vi "TLB Native Dynamic Events ver 0.25.vi"() -> ()   [LabVIEW 2018] (continued)
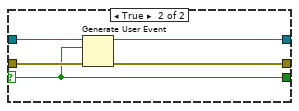
[diagram p2: hidden frame]
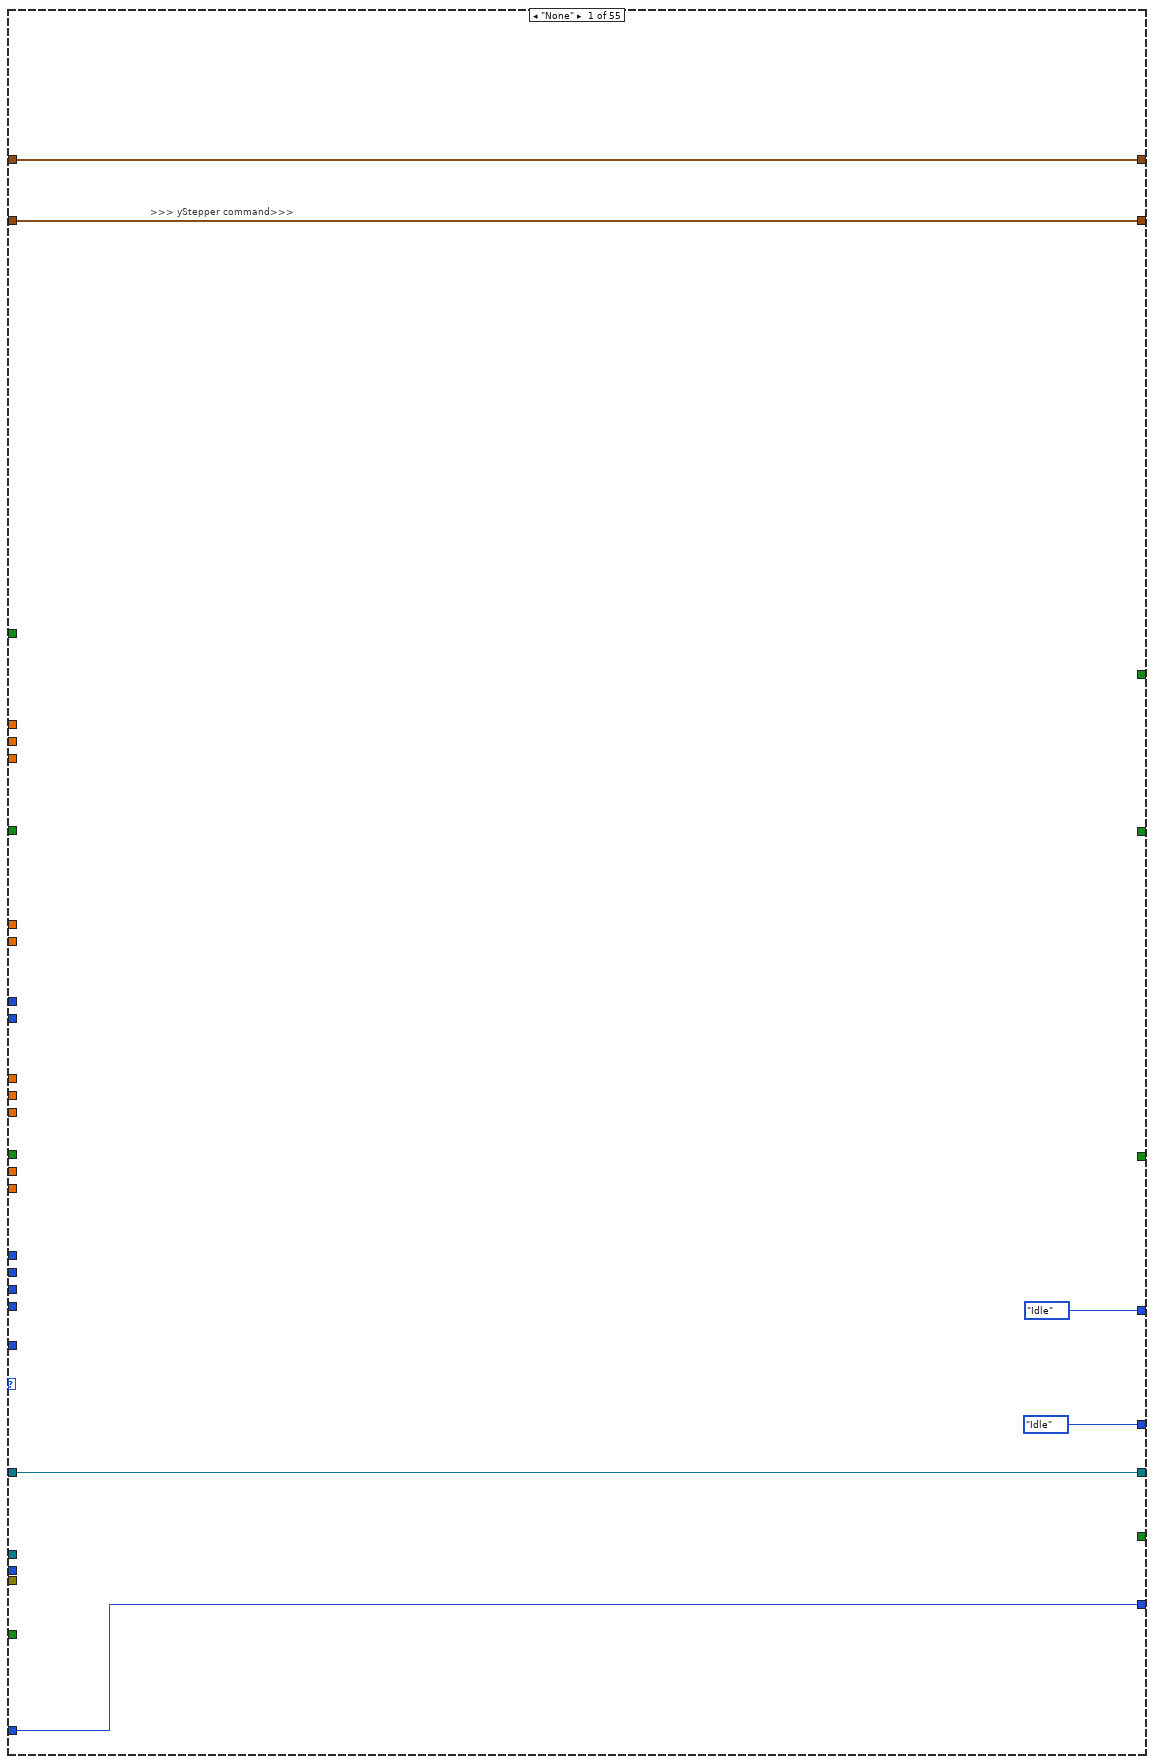
[diagram p5: hidden frame]
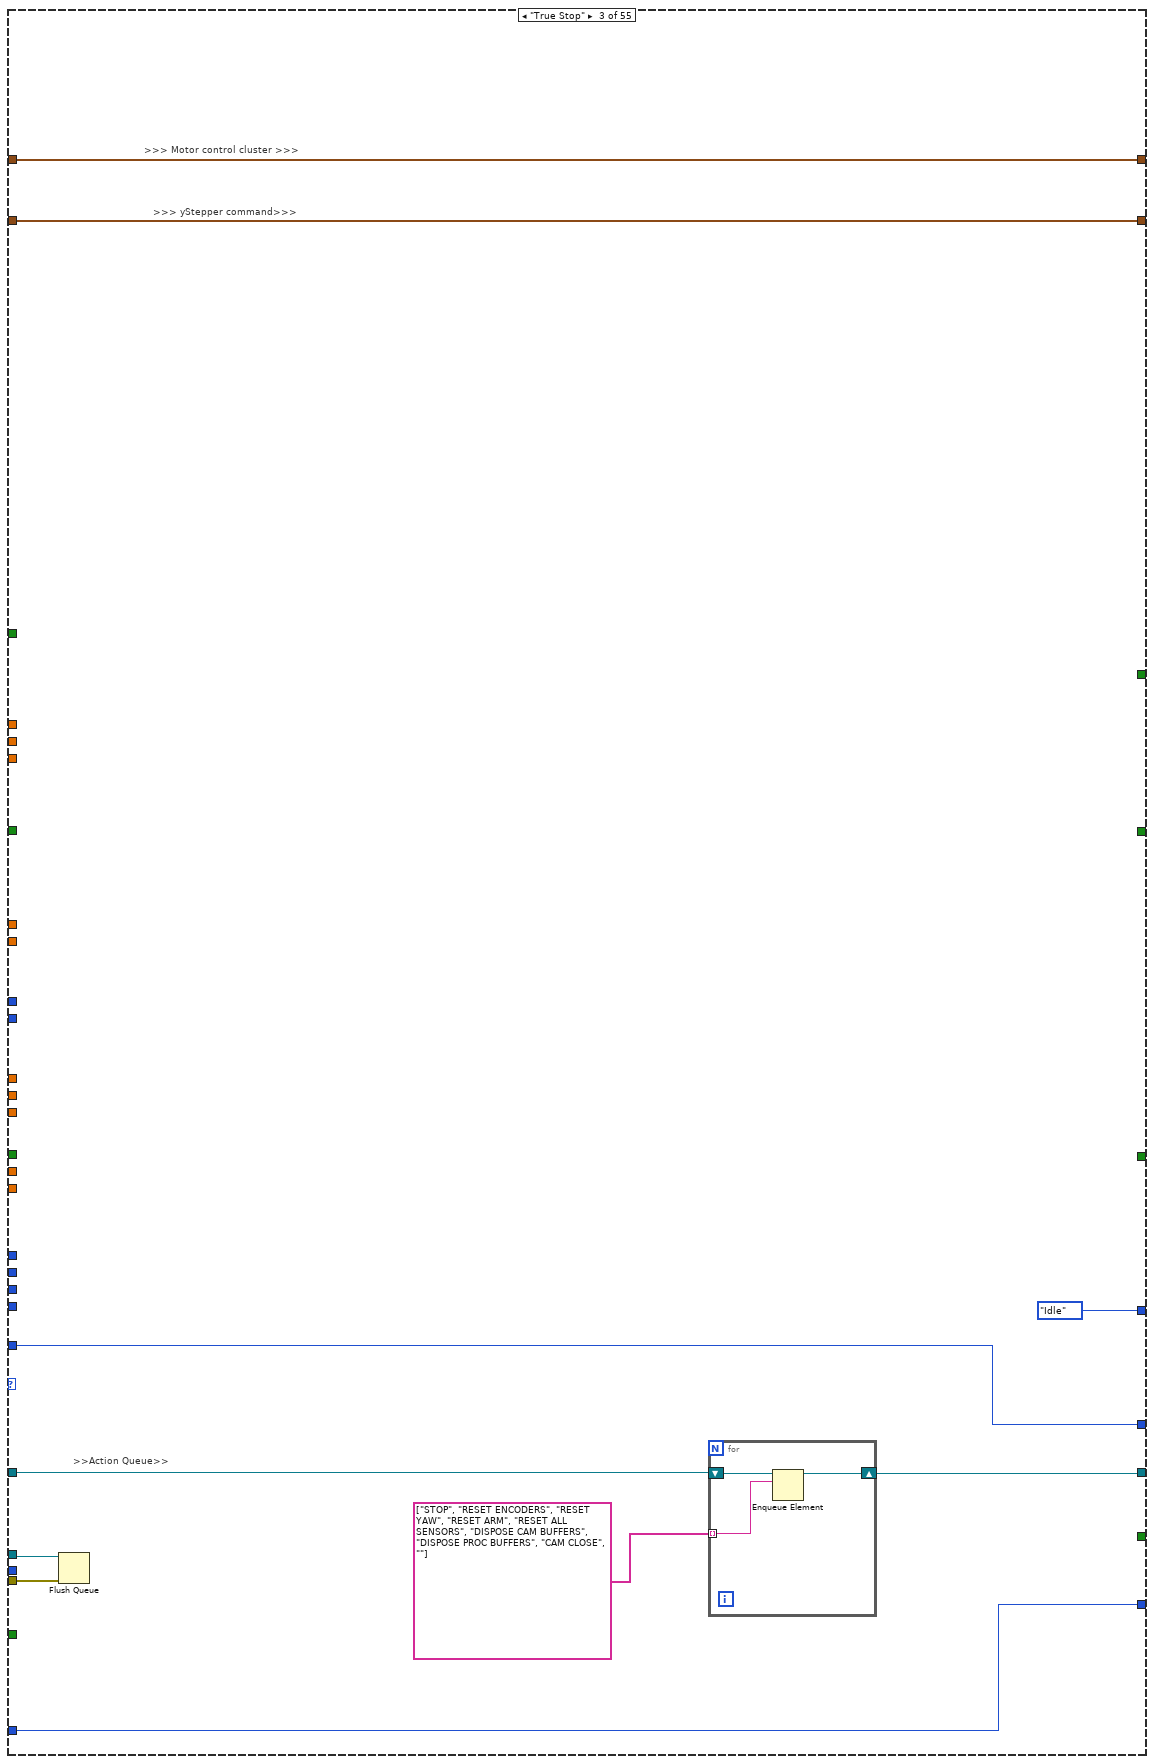
[diagram p6: hidden frame]
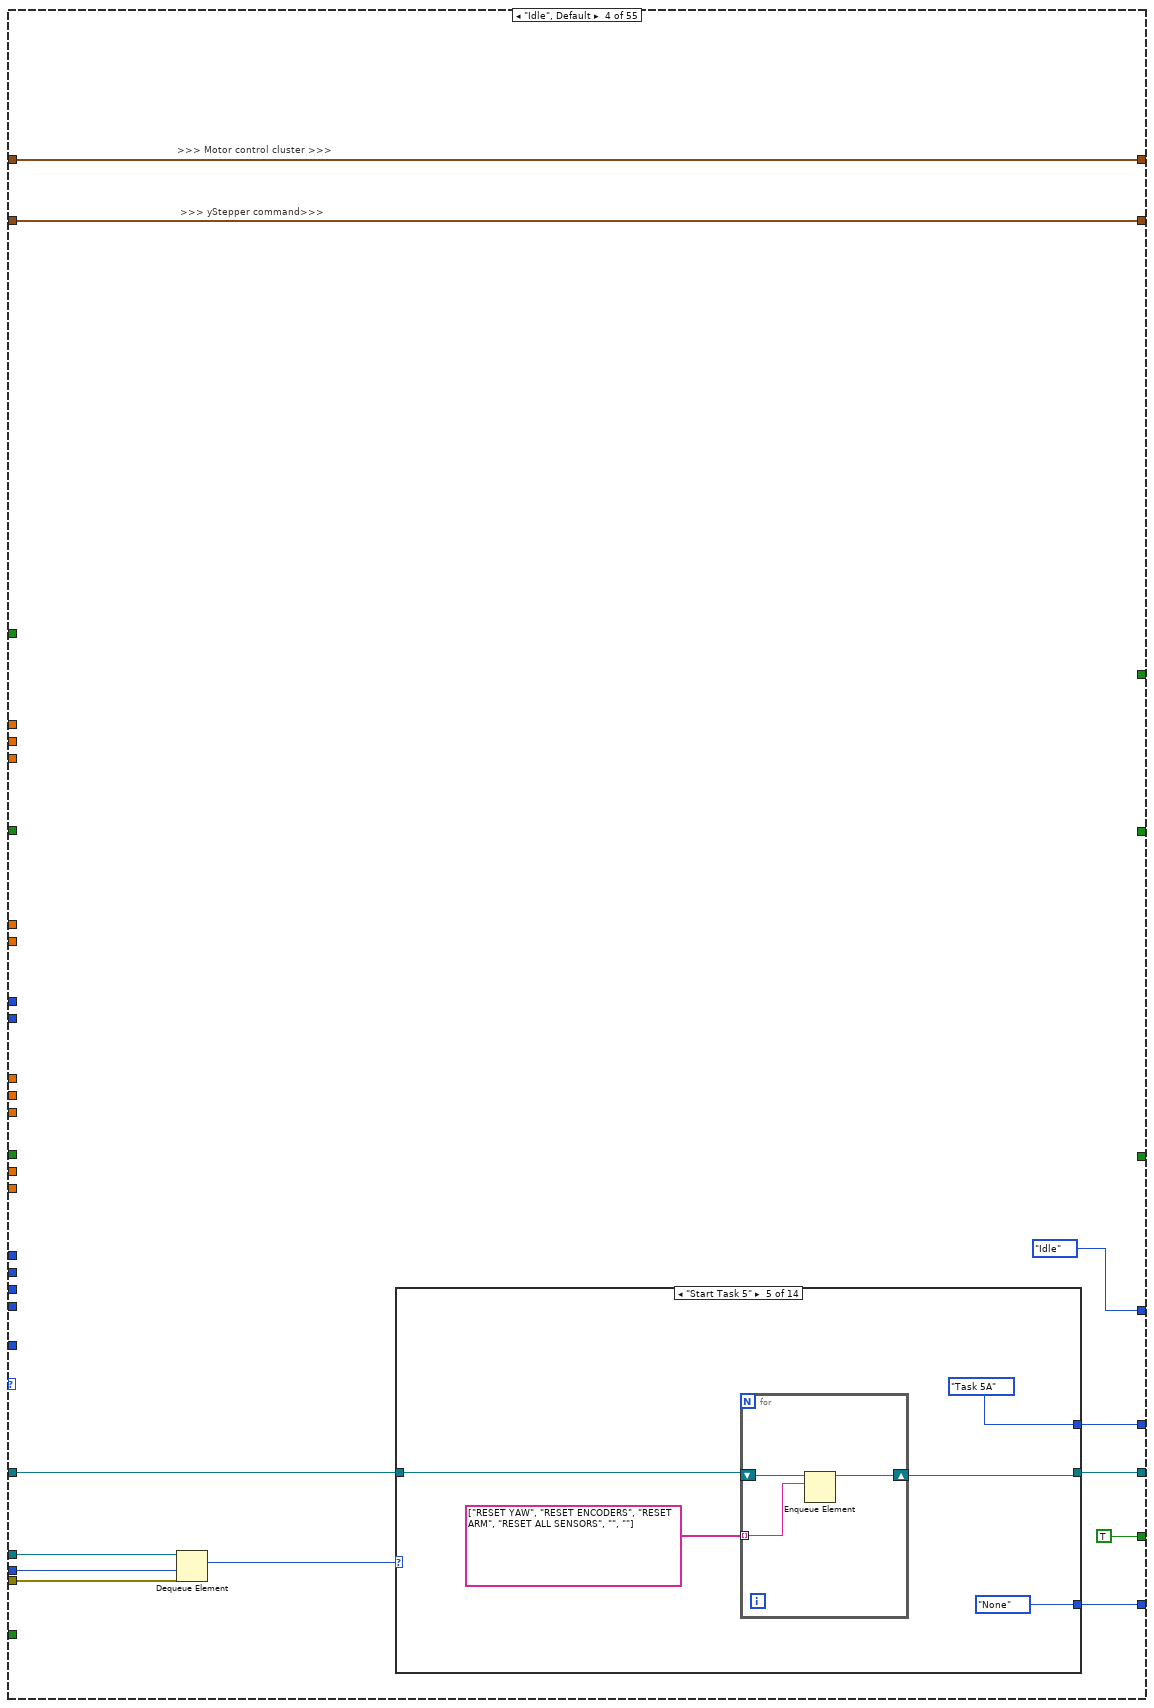
[diagram p7: hidden frame]
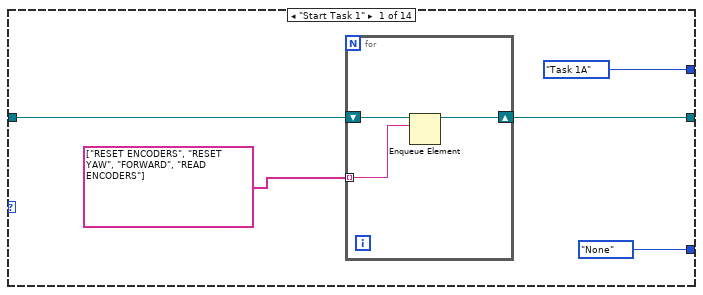
[diagram p8: hidden frame]
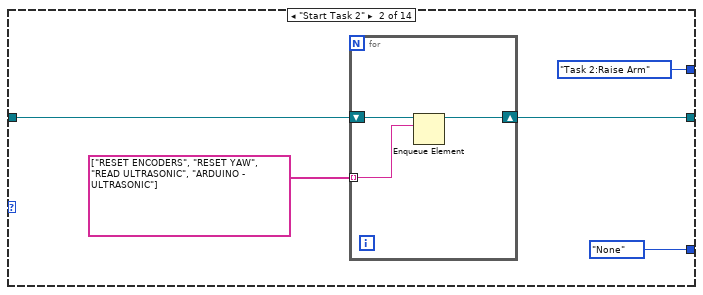
[diagram p9: hidden frame]
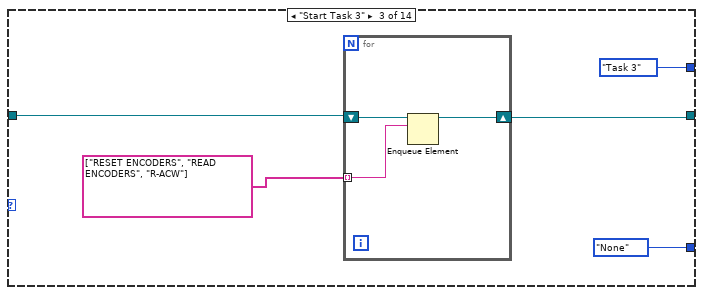
[diagram p10: hidden frame]
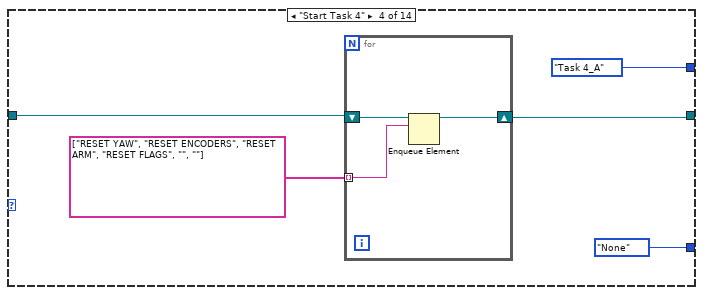
[diagram p11: hidden frame]
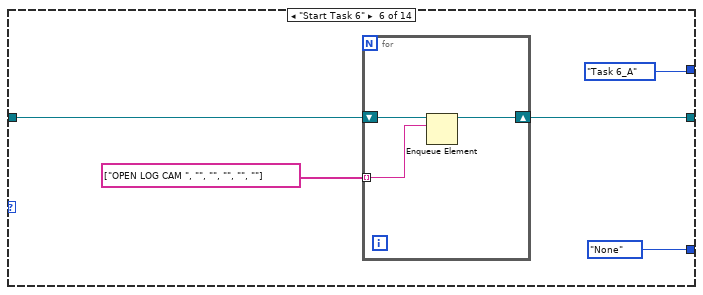
[diagram p12: hidden frame]
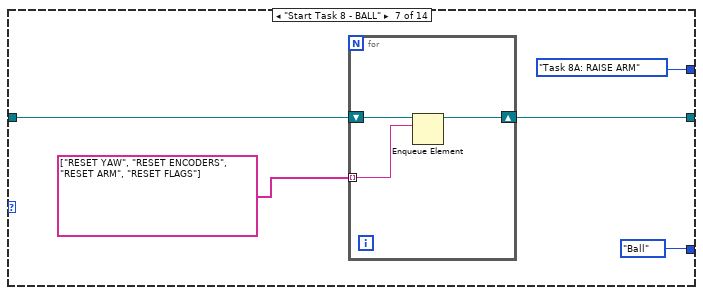
[diagram p13: hidden frame]
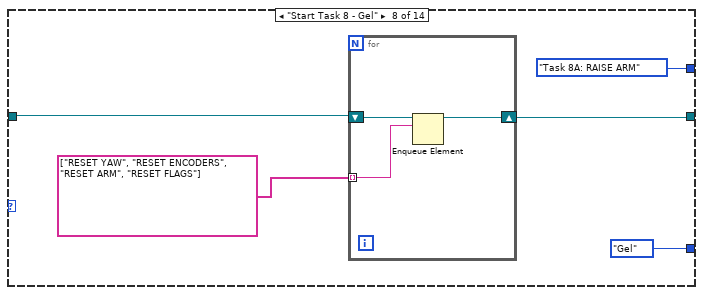
[diagram p14: hidden frame]
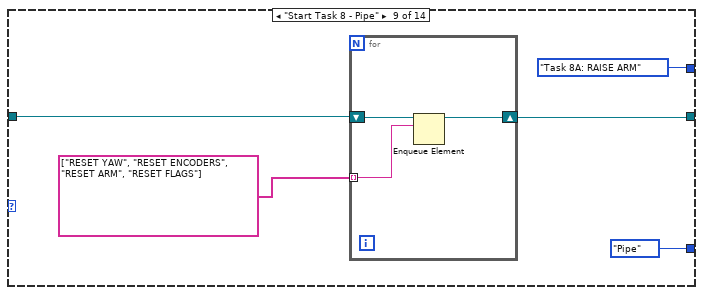
[diagram p15: hidden frame]
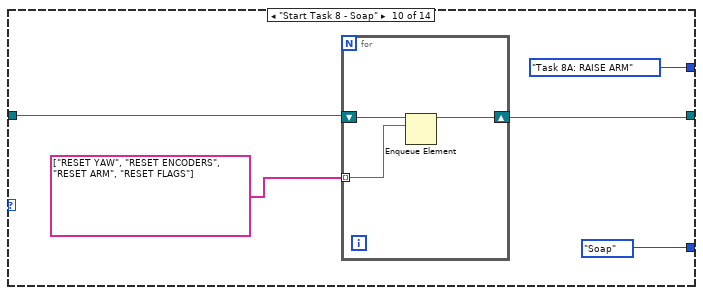
[diagram p16: hidden frame]
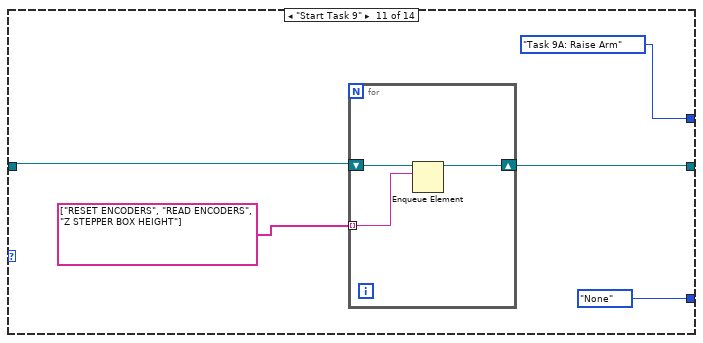
[diagram p17: hidden frame]
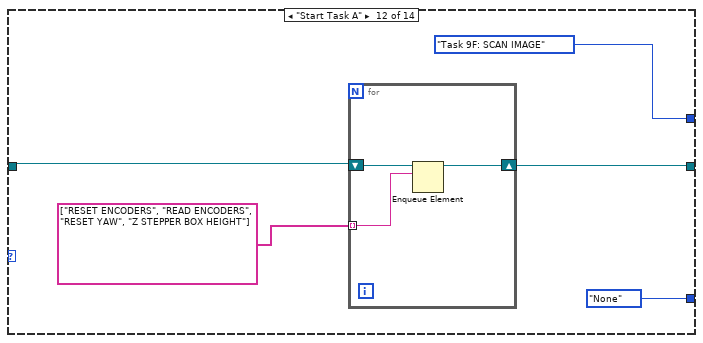
[diagram p18: hidden frame]
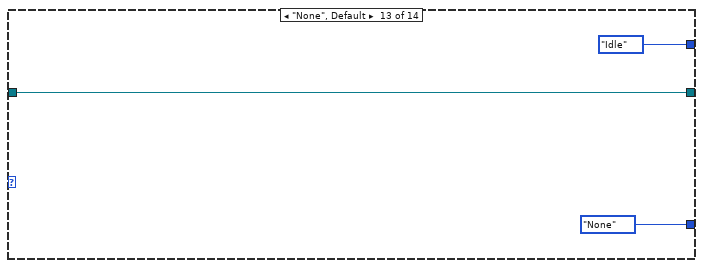
[diagram p19: hidden frame]
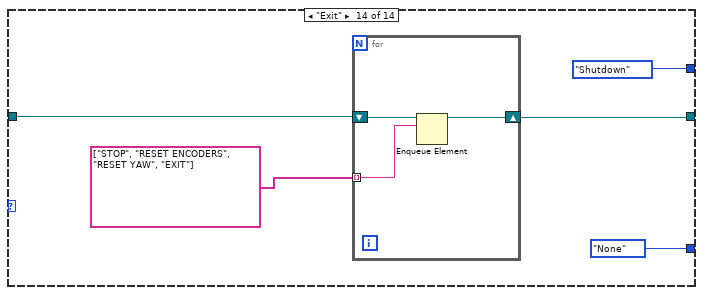
[diagram p20: hidden frame]
              tunnel: [w2327 State_Type_Definitions."True Stop" ("Enum")] -> w2311
              tunnel: w2309 -> [w2319 _]
              tunnel: w2313 -> [w2326 w2343]
              tunnel: [w2325 w2344] -> w2312
              tunnel: [State_Type_Definitions."Idle" ("Enum") State_Type_Definitions."Shutdown" ("Enum")] -> w2310
              frame "Start Task 1", Default {
                n755 = case shown="True" w2320 {
                  tunnel: w2326 -> [w2330 w2337]
                  tunnel: [w2331 w2336] -> w2325
                  frame False {
                    n756 = for {
                      tunnel: string[] ["START TIMER", "CAM ACQ", ""] ("element") -> [w2332] mode=indexing
                      shift-right: [w2334] -> w2331
                      shift-left: w2330 -> [w2333]
                      n757 = Enqueue Element(queue=w2333, element=w2332) -> (queue out=w2334:refnum<queue>)  [unwired: 2 in, 2 out]
                    }
                  }
                  frame True {
                    n758 = for {
                      shift-right: [w2339] -> w2336
                      shift-left: w2337 -> [w2340]
                      tunnel: string[] ["CLOSE CAM", "SET TIMER 5", "", "", "", ""] -> [w2338] mode=indexing
                      n759 = Enqueue Element(queue=w2340, element=w2338) -> (queue out=w2339:refnum<queue>)  [unwired: 2 in, 2 out]
                    }
                  }
                }
                n760 = Or(x=w2320, y=w2319) -> (x .or. y?=w2318:bool)
                n761 = Select(t=State_Type_Definitions."True Stop" ("Enum"), s=w2319, f=State_Type_Definitions."Task 9J: PROCESS COLOUR" ("Enum")) -> (s? t:f=w2321:T16)
                n762 = Select(t=w2321, s=w2318, f=State_Type_Definitions."Task 9I: SCAN IMAGE" ("Enum")) -> (s? t:f=w2327:T16)
              }
              frame "Exit" {
                n763 = for {
                  shift-right: [w2347] -> w2344
                  shift-left: w2343 -> [w2348]
                  tunnel: string[] ["STOP", "RESET ENCODERS", "RESET YAW", "ARDUINO MODE 0"] -> [w2346] mode=indexing
                  n764 = Enqueue Element(queue=w2348, element=w2346) -> (queue out=w2347:refnum<queue>)  [unwired: 2 in, 2 out]
                }
              }
            }
          }
          frame "Task 9J: PROCESS COLOUR" {
            # ">> Item Selection Bias >>"
            n765 = Dequeue Element(queue=w2354, timeout in ms (-1)=w2355, error in (no error)=w2356) -> (element=w2358:T8)  [unwired: 3 out]
            n766 = case shown="\"Start Task 1\", Default" w2358 {
              tunnel: w2349 -> [w2364 _]
              tunnel: [w2371 State_Type_Definitions."True Stop" ("Enum")] -> w2352
              tunnel: w2357 -> [w2363 _]
              tunnel: w2353 -> [w2370 w2387]
              tunnel: [w2369 w2388] -> w2351
              tunnel: [State_Type_Definitions."Idle" ("Enum") State_Type_Definitions."Shutdown" ("Enum")] -> w2350
              frame "Start Task 1", Default {
                n767 = case shown="True" w2364 {
                  tunnel: w2370 -> [w2374 w2381]
                  tunnel: [w2375 w2380] -> w2369
                  frame False {
                    n768 = for {
                      tunnel: string[] ["START TIMER", "COLOUR PROCESSING", ""] ("element") -> [w2376] mode=indexing
                      shift-right: [w2378] -> w2375
                      shift-left: w2374 -> [w2377]
                      n769 = Enqueue Element(queue=w2377, element=w2376) -> (queue out=w2378:refnum<queue>)  [unwired: 2 in, 2 out]
                    }
                  }
                  frame True {
                    n770 = for {
                      shift-right: [w2383] -> w2380
                      shift-left: w2381 -> [w2384]
                      tunnel: string[] ["CLOSE CAM", "DISPOSE BUFFERS", "RESET ENCODERS", "RESET YAW", "RESET FLAGS", ""] -> [w2382] mode=indexing
                      n771 = Enqueue Element(queue=w2384, element=w2382) -> (queue out=w2383:refnum<queue>)  [unwired: 2 in, 2 out]
                    }
                  }
                }
                n772 = Or(x=w2364, y=w2363) -> (x .or. y?=w2362:bool)
                n773 = Select(t=State_Type_Definitions."True Stop" ("Enum"), s=w2363, f=State_Type_Definitions."Task 9K: ROTATE 90 CW" ("Enum")) -> (s? t:f=w2365:T16)
                n774 = Select(t=w2365, s=w2362, f=State_Type_Definitions."Task 9J: PROCESS COLOUR" ("Enum")) -> (s? t:f=w2371:T16)
              }
              frame "Exit" {
                n775 = for {
                  shift-right: [w2391] -> w2388
                  shift-left: w2387 -> [w2392]
                  tunnel: string[] ["STOP", "RESET ENCODERS", "RESET YAW", "ARDUINO MODE 0"] -> [w2390] mode=indexing
                  n776 = Enqueue Element(queue=w2392, element=w2390) -> (queue out=w2391:refnum<queue>)  [unwired: 2 in, 2 out]
                }
              }
            }
          }
          frame "Task 9K: ROTATE 90 CW" {
            # ">>> Motor control cluster >>>"
            # ">>> yStepper command>>>"
            # ">> Item Selection Bias >>"
            n777 = Less?(x=w2396, y=-38.0) -> (x < y?=w2394:bool)
            n778 = Dequeue Element(queue=w2402, timeout in ms (-1)=w2401, error in (no error)=w2400) -> (element=w2404:T8)  [unwired: 3 out]
            n779 = case shown="\"Start Task 1\", Default" w2404 {
              tunnel: w2394 -> [w2410 _]
              tunnel: [w2417 State_Type_Definitions."True Stop" ("Enum")] -> w2398
              tunnel: w2399 -> [w2409 _]
              tunnel: w2403 -> [w2416 w2433]
              tunnel: [w2415 w2434] -> w2393
              tunnel: [State_Type_Definitions."Idle" ("Enum") State_Type_Definitions."Shutdown" ("Enum")] -> w2397
              frame "Start Task 1", Default {
                n780 = case shown="True" w2410 {
                  tunnel: w2416 -> [w2420 w2427]
                  tunnel: [w2421 w2426] -> w2415
                  frame False {
                    n781 = for {
                      tunnel: string[] ["READ ENCODERS", "R-CW"] ("element") -> [w2422] mode=indexing
                      shift-right: [w2424] -> w2421
                      shift-left: w2420 -> [w2423]
                      n782 = Enqueue Element(queue=w2423, element=w2422) -> (queue out=w2424:refnum<queue>)  [unwired: 2 in, 2 out]
                    }
                  }
                  frame True {
                    n783 = for {
                      shift-right: [w2429] -> w2426
                      shift-left: w2427 -> [w2430]
                      tunnel: string[] ["STOP", "RESET ENCODERS", "RESET FLAGS", "RESET YAW", "READ IR", "ARDUINO - ULTRASONIC"] -> [w2428] mode=indexing
                      n784 = Enqueue Element(queue=w2430, element=w2428) -> (queue out=w2429:refnum<queue>)  [unwired: 2 in, 2 out]
                    }
                  }
                }
                n785 = Or(x=w2410, y=w2409) -> (x .or. y?=w2408:bool)
                n786 = Select(t=State_Type_Definitions."True Stop" ("Enum"), s=w2409, f=State_Type_Definitions."Task 9L: MOVE FORWARD" ("Enum")) -> (s? t:f=w2411:T16)
                n787 = Select(t=w2411, s=w2408, f=State_Type_Definitions."Task 9K: ROTATE 90 CW" ("Enum")) -> (s? t:f=w2417:T16)
              }
              frame "Exit" {
                n788 = for {
                  shift-right: [w2437] -> w2434
                  shift-left: w2433 -> [w2438]
                  tunnel: string[] ["STOP", "RESET ENCODERS", "RESET YAW", "ARDUINO MODE 0"] -> [w2436] mode=indexing
                  n789 = Enqueue Element(queue=w2438, element=w2436) -> (queue out=w2437:refnum<queue>)  [unwired: 2 in, 2 out]
                }
              }
            }
          }
          frame "Task 9L: MOVE FORWARD" {
            w2451 = u8 50 ("y")
            # ">>> Motor control cluster >>>"
            # ">>> yStepper command>>>"
            # ">> Item Selection Bias >>"
            n790 = Less?(x=w2453, y=w2451) -> (x < y?=w2446:bool)
            n791 = Dequeue Element(queue=w2457, timeout in ms (-1)=w2456, error in (no error)=w2455) -> (element=w2461:T8)  [unwired: 3 out]
            n792 = Less?(x=w2452, y=w2451) -> (x < y?=w2447:bool)
            n793 = And(x=w2447, y=w2446) -> (x .and. y?=w2439:bool)
            n794 = Less Or Equal?(x=w2450, y=15.0) -> (x <= y?=w2445:bool)
            n795 = Greater?(x=w2444, y=100.0) -> (0:w2443:bool)
            n796 = Or(x=w2445, y=w2439) -> (x .or. y?=w2441:bool)
            n797 = And(x=w2443, y=w2441) -> (x .and. y?=w2442:bool)
            n798 = case shown="\"Start Task 1\", Default" w2461 {
              tunnel: w2442 -> [w2467 _]
              tunnel: [w2474 State_Type_Definitions."True Stop" ("Enum")] -> w2459
              tunnel: w2454 -> [w2466 _]
              tunnel: w2458 -> [w2473 w2490]
              tunnel: [w2472 w2491] -> w2448
              tunnel: [State_Type_Definitions."Idle" ("Enum") State_Type_Definitions."Shutdown" ("Enum")] -> w2460
              frame "Start Task 1", Default {
                n799 = case shown="True" w2467 {
                  tunnel: w2473 -> [w2477 w2484]
                  tunnel: [w2478 w2483] -> w2472
                  frame False {
                    n800 = for {
                      tunnel: string[] ["READ IR", "FORWARD", "READ NAVX", "READ ENCODERS"] ("element") -> [w2479] mode=indexing
                      shift-right: [w2481] -> w2478
                      shift-left: w2477 -> [w2480]
                      n801 = Enqueue Element(queue=w2480, element=w2479) -> (queue out=w2481:refnum<queue>)  [unwired: 2 in, 2 out]
                    }
                  }
                  frame True {
                    n802 = for {
                      shift-right: [w2486] -> w2483
                      shift-left: w2484 -> [w2487]
                      tunnel: string[] ["STOP", "RESET ENCODERS", "RESET FLAGS", "RESET YAW", "", ""] -> [w2485] mode=indexing
                      n803 = Enqueue Element(queue=w2487, element=w2485) -> (queue out=w2486:refnum<queue>)  [unwired: 2 in, 2 out]
                    }
                  }
                }
                n804 = Or(x=w2467, y=w2466) -> (x .or. y?=w2465:bool)
                n805 = Select(t=State_Type_Definitions."True Stop" ("Enum"), s=w2466, f=State_Type_Definitions."True Stop" ("Enum")) -> (s? t:f=w2468:T16)
                n806 = Select(t=w2468, s=w2465, f=State_Type_Definitions."Task 9L: MOVE FORWARD" ("Enum")) -> (s? t:f=w2474:T16)
              }
              frame "Exit" {
                n807 = for {
                  shift-right: [w2494] -> w2491
                  shift-left: w2490 -> [w2495]
                  tunnel: string[] ["STOP", "RESET ENCODERS", "RESET YAW", "ARDUINO MODE 0"] -> [w2493] mode=indexing
                  n808 = Enqueue Element(queue=w2495, element=w2493) -> (queue out=w2494:refnum<queue>)  [unwired: 2 in, 2 out]
                }
              }
            }
          }
          frame "Task 9M: MOVE RIGHT" {
            # ">> Item Selection Bias >>"
            n809 = Dequeue Element(queue=w2500, timeout in ms (-1)=w2499, error in (no error)=w2498) -> (element=w2505:T8)  [unwired: 3 out]
            n810 = case shown="\"Start Task 1\", Default" w2505 {
              tunnel: w2496 -> [w2511 _]
              tunnel: [w2518 State_Type_Definitions."True Stop" ("Enum")] -> w2503
              tunnel: w2497 -> [w2510 _]
              tunnel: w2501 -> [w2517 w2534]
              tunnel: [w2516 w2535] -> w2502
              tunnel: [State_Type_Definitions."Idle" ("Enum") State_Type_Definitions."Shutdown" ("Enum")] -> w2504
              frame "Start Task 1", Default {
                n811 = case shown="False" w2511 {
                  tunnel: w2517 -> [w2521 w2528]
                  tunnel: [w2522 w2527] -> w2516
                  frame False {
                    n812 = for {
                      tunnel: string[] ["READ LINE SENSOR", "READ NAVX", "RIGHT", "READ ENCODERS"] ("element") -> [w2523] mode=indexing
                      shift-right: [w2525] -> w2522
                      shift-left: w2521 -> [w2524]
                      n813 = Enqueue Element(queue=w2524, element=w2523) -> (queue out=w2525:refnum<queue>)  [unwired: 2 in, 2 out]
                    }
                  }
                  frame True {
                    n814 = for {
                      shift-right: [w2530] -> w2527
                      shift-left: w2528 -> [w2531]
                      tunnel: string[] ["STOP", "RESET ENCODERS", "RESET YAW", "OPEN LIFE CAM", "SET TIMER 2", "RESET FLAGS"] -> [w2529] mode=indexing
                      n815 = Enqueue Element(queue=w2531, element=w2529) -> (queue out=w2530:refnum<queue>)  [unwired: 2 in, 2 out]
                    }
                  }
                }
                n816 = Or(x=w2511, y=w2510) -> (x .or. y?=w2509:bool)
                n817 = Select(t=State_Type_Definitions."True Stop" ("Enum"), s=w2510, f=State_Type_Definitions."Task 9N: SCAN IMAGE" ("Enum")) -> (s? t:f=w2512:T16)
                n818 = Select(t=w2512, s=w2509, f=State_Type_Definitions."Task 9M: MOVE RIGHT" ("Enum")) -> (s? t:f=w2518:T16)
              }
              frame "Exit" {
                n819 = for {
                  shift-right: [w2538] -> w2535
                  shift-left: w2534 -> [w2539]
                  tunnel: string[] ["STOP", "RESET ENCODERS", "RESET YAW", "ARDUINO MODE 0"] -> [w2537] mode=indexing
                  n820 = Enqueue Element(queue=w2539, element=w2537) -> (queue out=w2538:refnum<queue>)  [unwired: 2 in, 2 out]
                }
              }
            }
          }
          frame "Task 9N: SCAN IMAGE" {
            # ">> Manual override >>"
            n821 = Dequeue Element(queue=w2548, timeout in ms (-1)=w2547, error in (no error)=w2546) -> (element=w2549:T8)  [unwired: 3 out]
            n822 = case shown="\"Start Task 1\", Default" w2549 {
              tunnel: [w2563 State_Type_Definitions."True Stop" ("Enum")] -> w2541
              tunnel: [w2561 w2579] -> w2540
              tunnel: w2544 -> [w2560 w2576]
              tunnel: w2545 -> [w2554 _]
              tunnel: [State_Type_Definitions."Idle" ("Enum") State_Type_Definitions."Shutdown" ("Enum")] -> w2542
              tunnel: w2543 -> [w2553 _]
              frame "Start Task 1", Default {
                # ">> WIill proceed to part ii if not manual override >>"
                # ">>If ENABLE or Trigger is set to true>>"
                n823 = Or(x=w2553, y=w2554) -> (x .or. y?=w2555:bool)
                n824 = case shown="False" w2553 {
                  tunnel: [w2566 w2572] -> w2561
                  tunnel: w2560 -> [w2565 w2571]
                  frame False {
                    n825 = for {
                      shift-right: [w2568] -> w2566
                      shift-left: w2565 -> [w2569]
                      tunnel: string[] ["CAM ACQ", "START TIMER"] ("element") -> [w2567] mode=indexing
                      n826 = Enqueue Element(queue=w2569, element=w2567) -> (queue out=w2568:refnum<queue>)  [unwired: 2 in, 2 out]
                    }
                  }
                  frame True {
                    n827 = for {
                      shift-right: [w2574] -> w2572
                      shift-left: w2571 -> [w2575]
                      tunnel: string[] ["CLOSE CAM", "SET TIMER 5", "", "", "", ""] -> [w2573] mode=indexing
                      n828 = Enqueue Element(queue=w2575, element=w2573) -> (queue out=w2574:refnum<queue>)  [unwired: 2 in, 2 out]
                    }
                  }
                }
                n829 = Select(t=State_Type_Definitions."True Stop" ("Enum"), s=w2554, f=State_Type_Definitions."Task 9O: PROCESS COLOUR" ("Enum")) -> (s? t:f=w2557:T16)
                n830 = Select(t=w2557, s=w2555, f=State_Type_Definitions."Task 9N: SCAN IMAGE" ("Enum")) -> (s? t:f=w2563:T16)
              }
              frame "Exit" {
                n831 = for {
                  shift-right: [w2582] -> w2579
                  shift-left: w2576 -> [w2583]
                  tunnel: string[] ["STOP", "RESET ENCODERS", "RESET YAW", ""] -> [w2581] mode=indexing
                  n832 = Enqueue Element(queue=w2583, element=w2581) -> (queue out=w2582:refnum<queue>)  [unwired: 2 in, 2 out]
                }
              }
            }
          }
          frame "Task 9O: PROCESS COLOUR" {
            # ">> Item Selection Bias >>"
            n833 = Dequeue Element(queue=w2591, timeout in ms (-1)=w2590, error in (no error)=w2589) -> (element=w2593:T8)  [unwired: 3 out]
            n834 = case shown="\"Start Task 1\", Default" w2593 {
              tunnel: w2584 -> [w2599 _]
              tunnel: [w2606 State_Type_Definitions."True Stop" ("Enum")] -> w2587
              tunnel: w2588 -> [w2598 _]
              tunnel: w2592 -> [w2605 w2622]
              tunnel: [w2604 w2623] -> w2586
              tunnel: [State_Type_Definitions."Idle" ("Enum") State_Type_Definitions."Shutdown" ("Enum")] -> w2585
              frame "Start Task 1", Default {
                n835 = case shown="False" w2599 {
                  tunnel: w2605 -> [w2609 w2616]
                  tunnel: [w2610 w2615] -> w2604
                  frame False {
                    n836 = for {
                      tunnel: string[] ["START TIMER", "COLOUR PROCESSING", ""] ("element") -> [w2611] mode=indexing
                      shift-right: [w2613] -> w2610
                      shift-left: w2609 -> [w2612]
                      n837 = Enqueue Element(queue=w2612, element=w2611) -> (queue out=w2613:refnum<queue>)  [unwired: 2 in, 2 out]
                    }
                  }
                  frame True {
                    n838 = for {
                      shift-right: [w2618] -> w2615
                      shift-left: w2616 -> [w2619]
                      tunnel: string[] ["CLOSE CAM", "DISPOSE BUFFERS", "RESET ENCODERS", "RESET YAW", "RESET FLAGS", ""] -> [w2617] mode=indexing
                      n839 = Enqueue Element(queue=w2619, element=w2617) -> (queue out=w2618:refnum<queue>)  [unwired: 2 in, 2 out]
                    }
                  }
                }
                n840 = Or(x=w2599, y=w2598) -> (x .or. y?=w2597:bool)
                n841 = Select(t=State_Type_Definitions."True Stop" ("Enum"), s=w2598, f=State_Type_Definitions."Task 9P: MOVE RIGHT" ("Enum")) -> (s? t:f=w2600:T16)
                n842 = Select(t=w2600, s=w2597, f=State_Type_Definitions."Task 9O: PROCESS COLOUR" ("Enum")) -> (s? t:f=w2606:T16)
              }
              frame "Exit" {
                n843 = for {
                  shift-right: [w2626] -> w2623
                  shift-left: w2622 -> [w2627]
                  tunnel: string[] ["STOP", "RESET ENCODERS", "RESET YAW", "ARDUINO MODE 0"] -> [w2625] mode=indexing
                  n844 = Enqueue Element(queue=w2627, element=w2625) -> (queue out=w2626:refnum<queue>)  [unwired: 2 in, 2 out]
                }
              }
            }
          }
          frame "Task 9P: MOVE RIGHT" {
            # ">> Item Selection Bias >>"
            n845 = Dequeue Element(queue=w2633, timeout in ms (-1)=w2632, error in (no error)=w2631) -> (element=w2641:T8)  [unwired: 3 out]
            n846 = Greater?(x=w2629, y=50.0) -> (0:w2639:bool)
            n847 = And(x=w2628, y=w2639) -> (x .and. y?=w2640:bool)
            n848 = case shown="\"Start Task 1\", Default" w2641 {
              tunnel: w2640 -> [w2647 _]
              tunnel: [w2654 State_Type_Definitions."True Stop" ("Enum")] -> w2636
              tunnel: w2630 -> [w2646 _]
              tunnel: w2634 -> [w2653 w2670]
              tunnel: [w2652 w2671] -> w2635
              tunnel: [State_Type_Definitions."Idle" ("Enum") State_Type_Definitions."Shutdown" ("Enum")] -> w2637
              frame "Start Task 1", Default {
                n849 = case shown="False" w2647 {
                  tunnel: w2653 -> [w2657 w2664]
                  tunnel: [w2658 w2663] -> w2652
                  frame False {
                    n850 = for {
                      tunnel: string[] ["READ LINE SENSOR", "READ NAVX", "RIGHT", "READ ENCODERS"] ("element") -> [w2659] mode=indexing
                      shift-right: [w2661] -> w2658
                      shift-left: w2657 -> [w2660]
                      n851 = Enqueue Element(queue=w2660, element=w2659) -> (queue out=w2661:refnum<queue>)  [unwired: 2 in, 2 out]
                    }
                  }
                  frame True {
                    n852 = for {
                      shift-right: [w2666] -> w2663
                      shift-left: w2664 -> [w2667]
                      tunnel: string[] ["STOP", "RESET ENCODERS", "RESET YAW", "OPEN LIFE CAM", "SET TIMER 2", "RESET FLAGS"] -> [w2665] mode=indexing
                      n853 = Enqueue Element(queue=w2667, element=w2665) -> (queue out=w2666:refnum<queue>)  [unwired: 2 in, 2 out]
                    }
                  }
                }
                n854 = Or(x=w2647, y=w2646) -> (x .or. y?=w2645:bool)
                n855 = Select(t=State_Type_Definitions."True Stop" ("Enum"), s=w2646, f=State_Type_Definitions."Task 9Q: SCAN IMAGE" ("Enum")) -> (s? t:f=w2648:T16)
                n856 = Select(t=w2648, s=w2645, f=State_Type_Definitions."Task 9P: MOVE RIGHT" ("Enum")) -> (s? t:f=w2654:T16)
              }
              frame "Exit" {
                n857 = for {
                  shift-right: [w2674] -> w2671
                  shift-left: w2670 -> [w2675]
                  tunnel: string[] ["STOP", "RESET ENCODERS", "RESET YAW", "ARDUINO MODE 0"] -> [w2673] mode=indexing
                  n858 = Enqueue Element(queue=w2675, element=w2673) -> (queue out=w2674:refnum<queue>)  [unwired: 2 in, 2 out]
                }
              }
            }
          }
          frame "Task 9Q: SCAN IMAGE" {
            # ">> Manual override >>"
            n859 = Dequeue Element(queue=w2684, timeout in ms (-1)=w2683, error in (no error)=w2682) -> (element=w2685:T8)  [unwired: 3 out]
            n860 = case shown="\"Start Task 1\", Default" w2685 {
              tunnel: [w2699 State_Type_Definitions."True Stop" ("Enum")] -> w2677
              tunnel: [w2697 w2715] -> w2676
              tunnel: w2680 -> [w2696 w2712]
              tunnel: w2681 -> [w2690 _]
              tunnel: [State_Type_Definitions."Idle" ("Enum") State_Type_Definitions."Shutdown" ("Enum")] -> w2678
              tunnel: w2679 -> [w2689 _]
              frame "Start Task 1", Default {
                # ">> WIill proceed to part ii if not manual override >>"
                # ">>If ENABLE or Trigger is set to true>>"
                n861 = Or(x=w2689, y=w2690) -> (x .or. y?=w2691:bool)
                n862 = case shown="False" w2689 {
                  tunnel: [w2702 w2708] -> w2697
                  tunnel: w2696 -> [w2701 w2707]
                  frame False {
                    n863 = for {
                      shift-right: [w2704] -> w2702
                      shift-left: w2701 -> [w2705]
                      tunnel: string[] ["CAM ACQ", "START TIMER"] ("element") -> [w2703] mode=indexing
                      n864 = Enqueue Element(queue=w2705, element=w2703) -> (queue out=w2704:refnum<queue>)  [unwired: 2 in, 2 out]
                    }
                  }
                  frame True {
                    n865 = for {
                      shift-right: [w2710] -> w2708
                      shift-left: w2707 -> [w2711]
                      tunnel: string[] ["CLOSE CAM", "SET TIMER 5", "", "", "", ""] -> [w2709] mode=indexing
                      n866 = Enqueue Element(queue=w2711, element=w2709) -> (queue out=w2710:refnum<queue>)  [unwired: 2 in, 2 out]
                    }
                  }
                }
                n867 = Select(t=State_Type_Definitions."True Stop" ("Enum"), s=w2690, f=State_Type_Definitions."Task 9R: PROCESS COLOUR" ("Enum")) -> (s? t:f=w2693:T16)
                n868 = Select(t=w2693, s=w2691, f=State_Type_Definitions."Task 9Q: SCAN IMAGE" ("Enum")) -> (s? t:f=w2699:T16)
              }
              frame "Exit" {
                n869 = for {
                  shift-right: [w2718] -> w2715
                  shift-left: w2712 -> [w2719]
                  tunnel: string[] ["STOP", "RESET ENCODERS", "RESET YAW", ""] -> [w2717] mode=indexing
                  n870 = Enqueue Element(queue=w2719, element=w2717) -> (queue out=w2718:refnum<queue>)  [unwired: 2 in, 2 out]
                }
              }
            }
          }
          frame "Task 9R: PROCESS COLOUR" {
            # ">> Item Selection Bias >>"
            # ">>> Motor control cluster >>>"
            # ">>> yStepper command>>>"
            n871 = Dequeue Element(queue=w2725, timeout in ms (-1)=w2726, error in (no error)=w2727) -> (element=w2729:T8)  [unwired: 3 out]
            n872 = case shown="\"Start Task 1\", Default" w2729 {
              tunnel: w2723 -> [w2735 _]
              tunnel: [w2742 State_Type_Definitions."True Stop" ("Enum")] -> w2721
              tunnel: w2728 -> [w2734 _]
              tunnel: w2724 -> [w2741 w2758]
              tunnel: [w2740 w2759] -> w2720
              tunnel: [State_Type_Definitions."Idle" ("Enum") State_Type_Definitions."Shutdown" ("Enum")] -> w2722
              frame "Start Task 1", Default {
                n873 = case shown="False" w2735 {
                  tunnel: w2741 -> [w2745 w2752]
                  tunnel: [w2746 w2751] -> w2740
                  frame False {
                    n874 = for {
                      tunnel: string[] ["START TIMER", "COLOUR PROCESSING", ""] ("element") -> [w2747] mode=indexing
                      shift-right: [w2749] -> w2746
                      shift-left: w2745 -> [w2748]
                      n875 = Enqueue Element(queue=w2748, element=w2747) -> (queue out=w2749:refnum<queue>)  [unwired: 2 in, 2 out]
                    }
                  }
                  frame True {
                    n876 = for {
                      shift-right: [w2754] -> w2751
                      shift-left: w2752 -> [w2755]
                      tunnel: string[] ["CLOSE CAM", "DISPOSE BUFFERS", "RESET ENCODERS", "RESET YAW", "RESET FLAGS", ""] -> [w2753] mode=indexing
                      n877 = Enqueue Element(queue=w2755, element=w2753) -> (queue out=w2754:refnum<queue>)  [unwired: 2 in, 2 out]
                    }
                  }
                }
                n878 = Or(x=w2735, y=w2734) -> (x .or. y?=w2733:bool)
                n879 = Select(t=State_Type_Definitions."True Stop" ("Enum"), s=w2734, f=State_Type_Definitions."True Stop" ("Enum")) -> (s? t:f=w2736:T16)
                n880 = Select(t=w2736, s=w2733, f=State_Type_Definitions."Task 9R: PROCESS COLOUR" ("Enum")) -> (s? t:f=w2742:T16)
              }
              frame "Exit" {
                n881 = for {
                  shift-right: [w2762] -> w2759
                  shift-left: w2758 -> [w2763]
                  tunnel: string[] ["STOP", "RESET ENCODERS", "RESET YAW", "ARDUINO MODE 0"] -> [w2761] mode=indexing
                  n882 = Enqueue Element(queue=w2763, element=w2761) -> (queue out=w2762:refnum<queue>)  [unwired: 2 in, 2 out]
                }
              }
            }
          }
        }
        "Object Detection" <- w307
        "Ultrasonic sensors" <- w330
        "Encoder values" <- w319
        "Stepper position values" <- w303
        "NAVX Values" <- w301
        "IR Sensors" <- w293
        "Line sensors" <- w288
        "Time cluster" <- w299
      }
    }
    "Object recognition mode" <- w215
    "Front Ultrasonic obstruct" <- w212
    "Front IR obstruct" <- w211
    "Table IR obstruct" <- w210
    n883 = local write "Green LED"(w225) -> ()
  }
  n884 = while {
    stop <- w3528 stop-if-true
    n885 = call "MOTOR CONTROL WITH PID AE.vi"("AE Mode"=MOTOR_CONTROL_WITH_PID_AE_DATA_MODE_TYPE_DEF."Read from AE") -> ("Speed & distance"=→"Speed & distance":T13)  [unwired: 3 in]
    n886 = call "FGV Bool.vi"("Init/Read/Write State"=States_for_Action_Engine."Read") -> ("Output node"=w3528:bool)  [unwired: 2 in, 1 out]
    n887 = Wait (ms)(milliseconds to wait=u32 5) -> ()  [unwired: 1 out]
  }
  n888 = call <vilib>:"DIO Close.vi"("error in (no error)"=w22, "DIO Info In"=w25) -> ()  [unwired: 9 in, 1 out]
  n889 = call <vilib>:"DIO Close.vi"("error in (no error)"=w32, "DIO Info In"=w34) -> ()  [unwired: 9 in, 1 out]
  n890 = call <vilib>:"NavX Close.vi"("error in (no error)"=w9, "NavX Info In"=w8) -> ()  [unwired: 9 in, 1 out]
  n891 = call <vilib>:"DIO Close.vi"("error in (no error)"=w27, "DIO Info In"=w29) -> ()  [unwired: 9 in, 1 out]
  n892 = call <vilib>:"DIO Close.vi"("error in (no error)"=w16, "DIO Info In"=w17) -> ()  [unwired: 9 in, 1 out]
  n893 = call <vilib>:"DIO Close.vi"("error in (no error)"=w11, "DIO Info In"=w12) -> ()  [unwired: 9 in, 1 out]
  n894 = Merge Errors "Merge Errors"(w62, w61) -> (w44:errorcluster)
  n895 = Merge Errors(w48, w44) -> (w43:errorcluster)
  n896 = Destroy User Event(user event=w66, error in=w43) -> ()  [unwired: 1 out]
  n897 = Release Queue(queue=w39, error in (no error)=w43) -> (error out=→"Queue Errors":errorcluster)  [unwired: 1 in, 2 out]
  n898 = Release Queue(queue=w56, error in (no error)=w43) -> ()  [unwired: 1 in, 3 out]
  n899 = Destroy User Event(user event=w65, error in=w43) -> ()  [unwired: 1 out]
  n900 = Unregister For Events(event registration refnum=w57, error in=w43) -> ()  [unwired: 1 out]
